vi "HFRR ADV v042.vi"() -> ()   [LabVIEW 2025] (continued)
                n3163 = local read "TITTLE"() -> (w3926:string)
                n3164 = call-dynamic "Set Report Header Text.vi"("report in"=w3909, "center header text"=w3926, "error in (no error)"=w3908) -> ("report out"=w3947:refnum<class "NI_report.lvclass">, "error out"=w3946:errorcluster)  [unwired: 11 in]
                n3165 = for {
                  N: 1 -> [_]
                  tunnel: [w3985] -> w3933
                  tunnel: [w3984] -> w3932
                  tunnel: w3947 -> [w3983]
                  tunnel: w3946 -> [w3982]
                  n3166 = call-dynamic "New Report Line.vi"("report in"=w3983, "error in (no error)"=w3982) -> ("report out"=w3985:refnum<class "NI_report.lvclass">, "error out"=w3984:errorcluster)  [unwired: 12 in]
                }
                n3167 = for {
                  N: 2 -> [_]
                  tunnel: [w3977] -> w3939
                  tunnel: [w3976] -> w3938
                  tunnel: w3933 -> [w3975]
                  tunnel: w3932 -> [w3974]
                  n3168 = call-dynamic "New Report Line.vi"("report in"=w3975, "error in (no error)"=w3974) -> ("report out"=w3977:refnum<class "NI_report.lvclass">, "error out"=w3976:errorcluster)  [unwired: 12 in]
                }
                n3169 = for {
                  N: 25 -> [_]
                  tunnel: w3939 -> [w3973]
                  tunnel: w3938 -> [w3971]
                  tunnel: [w3972] -> w3942
                  tunnel: [w3970] -> w3941
                  n3170 = call-dynamic "Set Report Tab Width.vi"("report in"=w3973, "error in (no error)"=w3971) -> ("report out"=w3972:refnum<class "NI_report.lvclass">, "error out"=w3970:errorcluster)  [unwired: 12 in]
                }
                n3171 = control-ref of="Tab Control 9"() -> (w3937:refnum<vi>)
                n3172 = call-dynamic "Append Control Image to Report.vi"("report in"=w3942, "alignment (default)"=HTML_Report_Image_Alignment."ABSMIDDLE", "ctrl reference"=w3937, "error in (no error)"=w3941) -> ("report out"=w3936:refnum<class "NI_report.lvclass">, "error out"=w3935:errorcluster)  [unwired: 8 in, 2 out]
                n3173 = for {
                  N: 3 -> [_]
                  tunnel: [w3969] -> w3920
                  tunnel: [w3968] -> w3919
                  tunnel: w3936 -> [w3967]
                  tunnel: w3935 -> [w3966]
                  n3174 = call-dynamic "New Report Line.vi"("report in"=w3967, "error in (no error)"=w3966) -> ("report out"=w3969:refnum<class "NI_report.lvclass">, "error out"=w3968:errorcluster)  [unwired: 12 in]
                }
                n3175 = for {
                  N: 100 -> [_]
                  tunnel: w3920 -> [w3965]
                  tunnel: w3919 -> [w3963]
                  tunnel: [w3964] -> w3916
                  tunnel: [w3962] -> w3914
                  n3176 = call-dynamic "Set Report Tab Width.vi"("report in"=w3965, "error in (no error)"=w3963) -> ("report out"=w3964:refnum<class "NI_report.lvclass">, "error out"=w3962:errorcluster)  [unwired: 12 in]
                }
                n3177 = String To Path(string="C:\\LAB-IQ\\im\\Temp_resized.jpg") -> (path=w3906:path)
                n3178 = call-poly <vilib>:"Append Image to Report.vi"("report in"=w3916, "path or URL of image"=w3906, "error in (no error)"=w3914) -> ("report out"=w3915:refnum<class "NI_report.lvclass">, "error out"=w3913:errorcluster)  [unwired: 9 in, 2 out]
                n3179 = call-poly <vilib>:"Open HTML Report in Browser.vi"("report in"=w3915, "error in (no error)"=w3913) -> ("report out"=w3950:refnum<class "NI_report.lvclass">, "error out"=w3949:errorcluster)  [unwired: 11 in, 1 out]
                n3180 = call-dynamic "Dispose Report.vi"("report in"=w3950, "error in (no error)"=w3949) -> ()  [unwired: 13 in, 1 out]
              }
              frame #2 {
              }
              frame #3 {
                n3181 = disable-structure shown="Disabled" {
                  frame Disabled {
                    n3182 = local read "String 10"() -> (w3990:string)
                    n3183 = Concatenate Strings("C:\\LAB-IQ-NXT\\Data\\" ("string"), w3990, ".jpg" ("string")) -> (w3988:string)
                    n3184 = String To Path(string=w3988) -> (path=w3987:path)
                    n3185 = Delete(path (use dialog)=w3987) -> ()  [unwired: 4 in, 3 out]
                  }
                  frame Enabled {
                  }
                }
                n3186 = local write "Print 2"(FALSE ("Print")) -> ()
              }
            }
          }
        }
      }
    }
    n3187 = Wait (ms)(milliseconds to wait=u32 50) -> ()  [unwired: 1 out]
    n3188 = Wait (ms)(milliseconds to wait=u32 50) -> ()  [unwired: 1 out]
    n3189 = local read "Quit"() -> (w2332:bool)
  }
  n3190 = VISA Close(VISA resource name=w43, error in (no error)=w42) -> ()  [unwired: 1 out]
  n3191 = while {
    stop <- w4141 stop-if-true
    n3192 = local read "Auto Start Test"() -> (w4139:bool)
    n3193 = local read "RUN"() -> (w4138:bool)
    n3194 = Wait (ms)(milliseconds to wait=u32 1000) -> ()  [unwired: 1 out]
    n3195 = Or(x=w4138, y=w4139) -> (x .or. y?=w4137:bool)
    n3196 = case shown="True" w4137 {
      frame False {
      }
      frame True {
        n3197 = local read "LVDT STROKE Actual"() -> (w4142:dbl)
        n3198 = In Range and Coerce(upper limit=1.2, x=w4142, lower limit=0.6) -> (In Range?=w4145:bool)  [unwired: 1 out]
        n3199 = call-poly <vilib>:"Random Number (Range).vi"("lower bound (0)"=0.998 ("upper bound (100)"), "upper bound (100)"=1.003) -> ("number"=w4143:dbl)  [unwired: 9 in]
        n3200 = case shown="True" w4145 {
          tunnel: [w4150 w4151] -> w4144
          tunnel: w4143 -> [_ w4151]
          tunnel: w4142 -> [w4150 _]
          frame False {
          }
          frame True {
          }
        }
        "LVDT STROKE DISPLAY" <- w4144
      }
    }
    n3201 = local read "Quit"() -> (w4141:bool)
  }
  n3202 = while {
    tunnel: [w4168] -> w51
    shift-right: [w4161] -> _
    shift-left: 0.0 -> [w4164]
    shift-right: [w4160] -> _
    shift-left: 0.0 -> [w4163]
    shift-right: [w4159] -> _
    shift-left: 100.0 ("vc_cmd") -> [w4162]
    stop <- w4168 stop-if-true
    # "PID LOGIC"
    n3203 = local read "run test Calibration"() -> (w4156:bool)
    n3204 = local read "RUN"() -> (w4166:bool)
    n3205 = local read "Auto Start Temp"() -> (w4157:bool)
    n3206 = local read "Auto Start Test"() -> (w4165:bool)
    n3207 = local read "START TEMP"() -> (w4155:bool)
    n3208 = And(x=w4157, y=w4165) -> (x .and. y?=w4158:bool)
    n3209 = Or(x=w4166, y=w4158) -> (x .or. y?=w4167:bool)
    n3210 = And(x=w4167, y=w4155) -> (x .and. y?=w4154:bool)
    n3211 = And(x=w4156, y=w4155) -> (x .and. y?=w4153:bool)
    n3212 = Or(x=w4153, y=w4154) -> (x .or. y?=w4152:bool)
    n3213 = Wait (ms)(milliseconds to wait="milliseconds to wait") -> ()  [unwired: 1 out]
    n3214 = case shown="True" w4152 {
      tunnel: [400.0 ("out_vc_cmd") w4187] -> w4159
      tunnel: [w4171 w4189] -> w4160
      tunnel: [w4171 w4188] -> w4161
      tunnel: w4164 -> [_ w4178]
      tunnel: w4163 -> [_ w4177]
      tunnel: w4162 -> [_ w4176]
      tunnel: w4156 -> [_ w4172]
      frame False {
        w4171 = 0.0 ("error_out")
      }
      frame True {
        n3215 = case shown="True" w4172 {
          tunnel: [w4196 1.0] -> w4174
          frame False {
            n3216 = local read "Set Strk"() -> (w4195:dbl)
            n3217 = Add(x=w4195, y="Add up Stroke") -> (x+y=w4196:dbl)
          }
          frame True {
          }
        }
        n3218 = local read "LVDT STROKE"() -> (w4173:dbl)
        n3219 = formula code="// Zero-Hardcode Explicit Positional-Form PID Engine\n// Inputs: target_stroke, measured_stroke, dt, prev_error, integral_accumulator_in, prev_vc_cmd\n//         kp, ki, kd, max_step_change, max_amplitude, min_amplitude, startup_cmd\n// Outputs: vc_cmd, error_out, out_error, integral_accumulator_out, out_vc_cmd\n\n// 1. Calculate Tracking Error\nfloat current_error = target_stroke - measured_stroke;\nerror_out = current_error;\n\n// 2. Compute Proportional Term\nfloat p_term = kp * current_error;\n\n// 3. Compute Derivative Term\nfloat d_term = 0.0;\nif (dt > 0.0) {\n    d_term = kd * ((current_error - prev_error) / dt);\n}\n\n// 4. Update and Accumulate Integral Term\nfloat current_integral = integral_accumulator_in + (current_error * dt);\nfloat i_term = ki * current_integral;\n\n// 5. Calculate Ideal Target Command (Anchored by startup baseline)\nfloat ideal_command = startup_cmd + p_term + i_term + d_term;\n\n// 6. Apply Loop Rate Limiting FIRST \n// (Forces the command to climb gradually from prev_vc_cmd instead of jumping straight to max)\nfloat raw_adjustment = ideal_command - prev_vc_cmd;\n\nif (raw_adjustment > max_step_change) {\n    raw_adjustment = max_step_change;\n} else if (raw_adjustment < -max_step_change) {\n    raw_adjustment = -max_step_change;\n}\n\nfloat next_vc_cmd = prev_vc_cmd + raw_adjustment;\n\n// 7. Anti-Windup Protection & Final Output Safety Safeguard Clamping\n// (Back-calculating based on what we are ACTUALLY outputting)\nif (next_vc_cmd > max_amplitude) {\n    float excess = next_vc_cmd - max_amplitude;\n    if (ki > 0.0) {\n        current_integral -= excess / ki;\n    }\n    next_vc_cmd = max_amplitude;\n} else if (next_vc_cmd < min_amplitude) {\n    float excess = next_vc_cmd - min_amplitude;\n    if (ki > 0.0) {\n        current_integral -= excess / ki;\n    }\n    next_vc_cmd = min_amplitude;\n}\n\n// 8. Map to Shift Registers for memory persistence\nvc_cmd = next_vc_cmd;\nout_error = current_error;                   \nintegral_accumulator_out = current_integral;  \nout_vc_cmd = next_vc_cmd;"("target_stroke"=w4174, "measured_stroke"=w4173, "dt"="dt", "integral_accumulator_in"=w4177, "prev_error"=w4178, "prev_vc_cmd"=w4176, "kp"="kp", "ki"="ki", "kd"="kd", "max_step_change"="max_step_change", "max_amplitude"="max_amplitude", "min_amplitude"="min_amplitude", "startup_cmd"="startup_cmd") -> ("vc_cmd"=w4193:dbl, "out_error"=w4188:dbl, "integral_accumulator_out"=w4189:dbl, "out_vc_cmd"=w4187:dbl)  [unwired: 1 out]
        "output Vpp" <- w4193
        n3220 = Number To Fractional String(number=w4193, precision (6)=i16 1) -> (F-format string=w4191:string)  [unwired: 2 in]
        n3221 = Concatenate Strings("DAC;" ("string"), w4191) -> (w4175:string)
        n3222 = local write "Due Write"(w4175) -> ()
        "prev_error" <- w4178
        "integral_accumulator_in" <- w4177
        "prev_vc_cmd" <- w4176
      }
    }
    n3223 = local read "Quit"() -> (w4168:bool)
  }
  n3224 = Or(x=w47, y=w46) -> (x .or. y?=w48:bool)
  n3225 = Or(x=w44, y=w48) -> (x .or. y?=w53:bool)
  n3226 = control-ref of="new picture"() -> ()  [unwired: 1 out]
  n3227 = Or(x=w56, y=w53) -> (x .or. y?=w50:bool)
  n3228 = Or(x=w50, y=w51) -> (x .or. y?=w45:bool)
  n3229 = while {
    tunnel: [w4198] -> w55
    i -> [w4205]
    stop <- w4198 stop-if-true
    n3230 = local read "Quit"() -> (w4198:bool)
    n3231 = Equal To 0?(x=w4205) -> (x = 0?=w4203:bool)
    n3232 = call "Elapsed Time3"("Time Target (s)"=45.0, "Auto Reset"=TRUE) -> ("Time has Elapsed"=w4202:bool)  [unwired: 10 in, 7 out]
    n3233 = Wait (ms)(milliseconds to wait=u32 50) -> ()  [unwired: 1 out]
    n3234 = Or(x=w4202, y=w4203) -> (x .or. y?=w4204:bool)
    n3235 = case shown="True" w4204 {
      frame False {
      }
      frame True {
        n3236 = call <vilib>:"System Exec.vi"("run minimized? (F)"=TRUE, "error in (no error)"="error in (no error)", "command line"="powercfg.exe -change -monitor-timeout-ac 0") -> ("error out"=w4216:errorcluster)  [unwired: 5 in, 3 out]
        n3237 = call <vilib>:"System Exec.vi"("run minimized? (F)"=TRUE, "error in (no error)"=w4216, "command line"="powercfg.exe -change -disk-timeout-ac 0") -> ("error out"=w4215:errorcluster)  [unwired: 5 in, 3 out]
        n3238 = call <vilib>:"System Exec.vi"("run minimized? (F)"=TRUE, "error in (no error)"=w4215, "command line"="powercfg.exe -change -standby-timeout-ac 0") -> ("error out"=w4214:errorcluster)  [unwired: 5 in, 3 out]
        n3239 = call <vilib>:"System Exec.vi"("run minimized? (F)"=TRUE, "error in (no error)"=w4214, "command line"="powercfg.exe -change -hibernate-timeout-ac 0") -> ("error out"=w4213:errorcluster)  [unwired: 5 in, 3 out]
        n3240 = call <vilib>:"Simple Error Handler.vi"("error in (no error)"=w4213) -> ("error out"=w4219:errorcluster)  [unwired: 4 in, 4 out]
        n3241 = call <vilib>:"Clear Errors.vi"("error in (no error)"=w4219) -> ("error out"=→"error out":errorcluster)  [unwired: 5 in, 1 out]
      }
    }
  }
  n3242 = Compound Arithmetic op=OR(w58, w45, w55) -> (w57:bool)
  n3243 = flat-sequence {
    tunnel: w57 -> [_]
    tunnel: [w4221] -> w27
    tunnel: w27 -> [_]
    frame #0 {
      n3244 = call "CLOSE CONNECTION.vi"() -> ("error out"=w4221:errorcluster)  [unwired: 11 in]
    }
    frame #1 {
      n3245 = Quit LabVIEW(quit? (T)=TRUE) -> ()
      n3246 = local write "Quit"(FALSE ("EXIT")) -> ()
    }
  }
  n3247 = property on="Heater Button" class="Bool (strict)"("Visible"=TRUE) -> ()  [unwired: 2 in, 2 out]
  n3248 = while {
    tunnel: [w4228] -> _
    i -> [w4228]
    stop <- w4224 stop-if-true
    # "Langauage selection"
    n3249 = Equal?(x="Lan flag", y=22.0) -> ()  [unwired: 1 out]
    n3250 = disable-structure shown="Disabled" {
      frame Disabled {
        n3251 = stacked-sequence {
          frame #0 {
            n3252 = case shown="\"Russian\"" "Language Selection" {
              tunnel: [0 1] -> w4230
              frame "English", Default {
              }
              frame "Russian" {
              }
            }
            n3253 = for {
              N: 130 -> [_]
              tunnel: "Table" -> [w4239]
              tunnel: w4230 -> [w4238]
              i -> [w4237]
              n3254 = Index Array(array=w4239, index (row)=w4237, index (col)=w4238) -> (element=w4236:string)
              n3255 = case shown="1" w4237 {
                tunnel: w4236 -> [w4240 w4241 _ w4242 w4243 w4244 w4245 w4246 w4247 w4248 w4249 w4250 w4251 w4252 w4253 w4254 w4255 w4256 w4257 w4258 w4259 w4260 w4261 w4262 w4263 w4264 w4265 w4266 w4267 _ _ w4268 w4269 w4270 w4271 w4272 w4273 w4282 w4289 w4296 w4303 w4307 w4310 w4313 w4315 w4317 w4318 w4319 w4320 w4321 w4322 w4323 w4324 w4325 w4326 w4327 w4328 w4329 w4330 w4331 w4332 w4333 w4334 w4335 w4336 w4337 w4338 w4339 w4340 w4341 w4342 w4343 w4344 w4345 w4346 w4347 w4348 w4349 w4350 w4351 w4352 w4353 w4354 w4355 w4356 w4357 w4358 w4359 w4360 w4361 w4362 w4363 w4364 w4365 w4366 w4367 w4368 w4369 w4370 w4371 w4372 w4373 w4374 w4375 w4376 _ w4377 w4378 w4379 w4380 w4381 w4382 w4383 w4384 w4385 w4386 w4387 w4388 w4389 _ w4390 w4391 w4392 w4393 w4394 w4395 _]
                frame 0 {
                  n3256 = local write "S"(w4240) -> ()
                }
                frame 1 {
                  n3257 = local write "S 2"(w4241) -> ()
                }
                frame 2 {
                }
                frame 3 {
                  n3258 = local write "S 4"(w4242) -> ()
                }
                frame 4 {
                  n3259 = property on="FILE" class="Str"("Caption.Text"=w4243) -> ()  [unwired: 2 in, 2 out]
                }
                frame 5 {
                  n3260 = property on="Fuel Discription :" class="Str"("Caption.Text"=w4244) -> ()  [unwired: 2 in, 2 out]
                }
                frame 6 {
                  n3261 = property on="Remarks :" class="Str"("Caption.Text"=w4245) -> ()  [unwired: 2 in, 2 out]
                }
                frame 7 {
                  n3262 = property on="Save & Continue" class="Bool (strict)"("Boolean Text.Text"=w4246) -> ()  [unwired: 2 in, 2 out]
                }
                frame 8 {
                }
                frame 9 {
                  n3263 = property on="Set Hz" class="DigNum (strict)"("Caption.Text"=w4248) -> ()  [unwired: 2 in, 2 out]
                }
                frame 10 {
                }
                frame 11 {
                  n3264 = property on="NORMAL LOAD" class="DigNum (strict)"("Caption.Text"=w4250) -> ()  [unwired: 2 in, 2 out]
                }
                frame 12 {
                }
                frame 13 {
                  n3265 = property on="Set Temp" class="DigNum (strict)"("Caption.Text"=w4252) -> ()  [unwired: 2 in, 2 out]
                }
                frame 14 {
                  n3266 = local write "S 15"(w4253) -> ()
                }
                frame 15 {
                  n3267 = property on="Set Rh" class="DigNum (strict)"("Caption.Text"=w4254) -> ()  [unwired: 2 in, 2 out]
                }
                frame 16 {
                }
                frame 17 {
                  n3268 = local write "S 18"(w4256) -> ()
                }
                frame 18 {
                  "String 17" <- w4257
                }
                frame 19 {
                  n3269 = property on="test time" class="DigNum (strict)"("Caption.Text"=w4258) -> ()  [unwired: 2 in, 2 out]
                }
                frame 20 {
                  "String 18" <- w4259
                  "String 22" <- w4259
                }
                frame 21 {
                  n3270 = property on="Elapsed time" class="DigNum (strict)"("Caption.Text"=w4260) -> ()  [unwired: 2 in, 2 out]
                }
                frame 22 {
                  n3271 = property on="Samplingtime 2" class="DigNum (strict)"("Caption.Text"=w4261) -> ()  [unwired: 2 in, 2 out]
                }
                frame 23 {
                  "String 21" <- w4262
                }
                frame 24 {
                  n3272 = property on="Countdown" class="DigNum (strict)"("Caption.Text"=w4263) -> ()  [unwired: 2 in, 2 out]
                }
                frame 25 {
                  n3273 = property on="Countdown 2" class="DigNum (strict)"("Caption.Text"=w4264) -> ()  [unwired: 2 in, 2 out]
                }
                frame 26 {
                  n3274 = property on="Engage" class="Bool (strict)"("Boolean Text.Text"=w4265) -> ()  [unwired: 2 in, 2 out]
                }
                frame 27 {
                  n3275 = property on="Boolean  4" class="Bool (strict)"("Boolean Text.Text"=w4266) -> ()  [unwired: 2 in, 2 out]
                }
                frame 28 {
                  n3276 = property on="Test \nStatus" class="Bool (strict)"("Boolean Text.Text"=w4267) -> ()  [unwired: 2 in, 2 out]
                }
                frame 29 {
                }
                frame 30 {
                }
                frame 31 {
                }
                frame 32 {
                  n3277 = property on="RSTCOF" class="Bool"("Boolean Text.Text"=w4269) -> ()  [unwired: 2 in, 2 out]
                  n3278 = property on="RST FF" class="Bool"("Boolean Text.Text"=w4269) -> ()  [unwired: 2 in, 2 out]
                  n3279 = property on="RST TEMP" class="Bool"("Boolean Text.Text"=w4269) -> ()  [unwired: 2 in, 2 out]
                  n3280 = property on="RSTV1 3" class="Bool"("Boolean Text.Text"=w4269) -> ()  [unwired: 2 in, 2 out]
                  n3281 = property on="rstv2" class="Bool"("Boolean Text.Text"=w4269) -> ()  [unwired: 2 in, 2 out]
                  n3282 = property on="RSTV1 2" class="Bool"("Boolean Text.Text"=w4269) -> ()  [unwired: 2 in, 2 out]
                  n3283 = property on="RST CP" class="Bool"("Boolean Text.Text"=w4269) -> ()  [unwired: 2 in, 2 out]
                }
                frame 33 {
                  "S 61" <- w4270
                }
                frame 34 {
                  "String 23" <- w4271
                }
                frame 35 {
                  n3284 = property on="Rh Before" class="DigNum (strict)"("Caption.Text"=w4272) -> ()  [unwired: 2 in, 2 out]
                }
                frame 36 {
                  n3285 = Match Pattern(string=w4273, regular expression=",") -> (before substring=→"bs":string, after substring=→"as":string)  [unwired: 1 in, 2 out]
                  n3286 = property on="Rh After" class="DigNum (strict)"("Caption.Text"=w4273) -> ()  [unwired: 2 in, 2 out]
                }
                frame 37 {
                  n3287 = Match Pattern(string=w4282, regular expression=",") -> (before substring=w4281:string, after substring=w4280:string)  [unwired: 1 in, 2 out]
                  "bs" <- w4281
                  "as" <- w4280
                  n3288 = Concatenate Strings(w4281, w4280) -> (w4277:string)
                  n3289 = property on="Humidity before test 2" class="DigNum (strict)"("Caption.Text"=w4277) -> ()  [unwired: 2 in, 2 out]
                  n3290 = Concatenate Strings(w4277, "=" ("string")) -> (w4278:string)
                  n3291 = local write "S 38"(w4278) -> ()
                }
                frame 38 {
                  n3292 = Match Pattern(string=w4289, regular expression=",") -> (before substring=w4288:string, after substring=w4287:string)  [unwired: 1 in, 2 out]
                  "bs" <- w4288
                  "as" <- w4287
                  n3293 = Concatenate Strings(w4288, w4287) -> (w4284:string)
                  n3294 = property on="Humidity after test 2" class="DigNum (strict)"("Caption.Text"=w4284) -> ()  [unwired: 2 in, 2 out]
                  n3295 = Concatenate Strings(w4284, "=" ("string")) -> (w4286:string)
                  n3296 = local write "S 39"(w4286) -> ()
                }
                frame 39 {
                  n3297 = Match Pattern(string=w4296, regular expression=",") -> (before substring=w4295:string, after substring=w4294:string)  [unwired: 1 in, 2 out]
                  "bs" <- w4295
                  "as" <- w4294
                  n3298 = Concatenate Strings(w4295, w4294) -> (w4291:string)
                  n3299 = property on="Temperature before test 2" class="DigNum (strict)"("Caption.Text"=w4291) -> ()  [unwired: 2 in, 2 out]
                  n3300 = Concatenate Strings(w4291, "=" ("string")) -> (→"String 34":string)
                }
                frame 40 {
                  n3301 = Match Pattern(string=w4303, regular expression=",") -> (before substring=w4302:string, after substring=w4301:string)  [unwired: 1 in, 2 out]
                  "bs" <- w4302
                  "as" <- w4301
                  n3302 = Concatenate Strings(w4302, w4301) -> (w4298:string)
                  n3303 = property on="Temperature after test 2" class="DigNum (strict)"("Caption.Text"=w4298) -> ()  [unwired: 2 in, 2 out]
                  n3304 = Concatenate Strings(w4298, "=" ("string")) -> (→"String 35":string)
                  n3305 = property on="Temperature after test" class="DigNum (strict)"("Caption.Text"=w4298) -> ()  [unwired: 2 in, 2 out]
                }
                frame 41 {
                  n3306 = property on="AVP 2" class="DigNum (strict)"("Caption.Text"=w4307) -> ()  [unwired: 2 in, 2 out]
                  n3307 = Concatenate Strings(w4307, "=" ("string")) -> (→"String 36":string)
                }
                frame 42 {
                  n3308 = property on="MWSD 2" class="DigNum (strict)"("Caption.Text"=w4310) -> ()  [unwired: 2 in, 2 out]
                  n3309 = Concatenate Strings(w4310, "=" ("string")) -> (→"String 37":string)
                }
                frame 43 {
                  n3310 = property on="HCF 2" class="DigNum (strict)"("Caption.Text"=w4313) -> ()  [unwired: 2 in, 2 out]
                  n3311 = Concatenate Strings(w4313, "=" ("string")) -> (→"String 38":string)
                }
                frame 44 {
                  n3312 = Concatenate Strings(w4315, "=" ("string")) -> (→"String 39":string)
                  n3313 = property on="WS1.4 2" class="DigNum (strict)"("Caption.Text"=w4315) -> ()  [unwired: 2 in, 2 out]
                }
                frame 45 {
                }
                frame 46 {
                  n3314 = local write "S 47"(w4318) -> ()
                }
                frame 47 {
                  n3315 = local write "S 48"(w4319) -> ()
                }
                frame 48 {
                  n3316 = local write "S 49"(w4320) -> ()
                }
                frame 49 {
                  n3317 = local write "S 50"(w4321) -> ()
                }
                frame 50 {
                  n3318 = local write "S 51"(w4322) -> ()
                }
                frame 51 {
                  n3319 = local write "S 52"(w4323) -> ()
                }
                frame 52 {
                  n3320 = local write "S 53"(w4324) -> ()
                }
                frame 53 {
                  n3321 = local write "S 54"(w4325) -> ()
                }
                frame 54 {
                  n3322 = local write "S 55"(w4326) -> ()
                }
                frame 55 {
                  n3323 = local write "S 56"(w4327) -> ()
                }
                frame 56 {
                  n3324 = local write "S 57"(w4328) -> ()
                }
                frame 57 {
                  n3325 = local write "S 58"(w4329) -> ()
                }
                frame 58 {
                  n3326 = local write "S 59"(w4330) -> ()
                }
                frame 59 {
                  n3327 = local write "S 60"(w4331) -> ()
                }
                frame 60 {
                  n3328 = local write "S 62"(w4332) -> ()
                }
                frame 61 {
                  n3329 = local write "S 63"(w4333) -> ()
                }
                frame 62 {
                  n3330 = local write "S 64"(w4334) -> ()
                }
                frame 63 {
                  n3331 = local write "S 65"(w4335) -> ()
                }
                frame 64 {
                  n3332 = local write "S 66"(w4336) -> ()
                }
                frame 65 {
                  n3333 = local write "S 67"(w4337) -> ()
                }
                frame 66 {
                  n3334 = local write "S 68"(w4338) -> ()
                }
                frame 67 {
                  n3335 = local write "S 69"(w4339) -> ()
                }
                frame 68 {
                  n3336 = local write "S 70"(w4340) -> ()
                }
                frame 69 {
                  n3337 = local write "S 71"(w4341) -> ()
                }
                frame 70 {
                  n3338 = local write "S 72"(w4342) -> ()
                }
                frame 71 {
                  n3339 = local write "S 73"(w4343) -> ()
                }
                frame 72 {
                  n3340 = local write "S 74"(w4344) -> ()
                }
                frame 73 {
                  n3341 = local write "S 75"(w4345) -> ()
                }
                frame 74 {
                  n3342 = local write "S 76"(w4346) -> ()
                }
                frame 75 {
                  n3343 = local write "S 77"(w4347) -> ()
                }
                frame 76 {
                  n3344 = local write "S 78"(w4348) -> ()
                }
                frame 77 {
                  n3345 = local write "S 79"(w4349) -> ()
                }
                frame 79 {
                  n3346 = property on="Sample Temperature ( °C )" class="XYGraph (strict)"("Y Scale.Name Label.Text"=w4350) -> ()  [unwired: 2 in, 2 out]
                }
                frame 80 {
                  n3347 = local write "S 81"(w4351) -> ()
                  n3348 = property on="Humidity ( %RH )" class="XYGraph (strict)"("Y Scale.Name Label.Text"=w4351) -> ()  [unwired: 2 in, 2 out]
                }
                frame 78 {
                  n3349 = property on="Air Temperature  ( °C )" class="XYGraph (strict)"("X Scale.Name Label.Text"=w4352) -> ()  [unwired: 2 in, 2 out]
                  n3350 = property on="Humidity ( %RH )" class="XYGraph (strict)"("X Scale.Name Label.Text"=w4352) -> ()  [unwired: 2 in, 2 out]
                  n3351 = property on="Sample Temperature ( °C )" class="XYGraph (strict)"("X Scale.Name Label.Text"=w4352) -> ()  [unwired: 2 in, 2 out]
                  n3352 = property on="Coefficient Of Friction" class="XYGraph (strict)"("X Scale.Name Label.Text"=w4352) -> ()  [unwired: 2 in, 2 out]
                }
                frame 81 {
                  n3353 = property on="Air Temperature  ( °C )" class="XYGraph (strict)"("Y Scale.Name Label.Text"=w4353) -> ()  [unwired: 2 in, 2 out]
                }
                frame 82 {
                  n3354 = local write "S 84"(w4354) -> ()
                }
                frame 83 {
                  n3355 = local write "S 85"(w4355) -> ()
                }
                frame 84 {
                  n3356 = local write "S 86"(w4356) -> ()
                }
                frame 85 {
                  n3357 = local write "S 87"(w4357) -> ()
                }
                frame 86 {
                  n3358 = local write "S 88"(w4358) -> ()
                }
                frame 87 {
                }
                frame 88 {
                  n3359 = local write "S 90"(w4360) -> ()
                }
                frame 89 {
                  n3360 = local write "S 91"(w4361) -> ()
                }
                frame 90 {
                  n3361 = local write "S 92"(w4362) -> ()
                }
                frame 91 {
                  n3362 = local write "S 93"(w4363) -> ()
                }
                frame 92 {
                  n3363 = local write "S 94"(w4364) -> ()
                }
                frame 93 {
                  n3364 = local write "S 95"(w4365) -> ()
                }
                frame 94 {
                  n3365 = local write "S 96"(w4366) -> ()
                }
                frame 95 {
                  n3366 = local write "S 97"(w4367) -> ()
                }
                frame 96 {
                  n3367 = local write "S 98"(w4368) -> ()
                }
                frame 97 {
                  n3368 = local write "S 99"(w4369) -> ()
                }
                frame 98 {
                  n3369 = local write "S 100"(w4370) -> ()
                }
                frame 99 {
                  n3370 = local write "S 101"(w4371) -> ()
                }
                frame 100 {
                  n3371 = local write "S 102"(w4372) -> ()
                }
                frame 101 {
                  n3372 = local write "S 103"(w4373) -> ()
                }
                frame 102 {
                  n3373 = local write "S 104"(w4374) -> ()
                }
                frame 103 {
                  n3374 = local write "S 105"(w4375) -> ()
                }
                frame 104 {
                  n3375 = local write "S 106"(w4376) -> ()
                }
                frame 105 {
                }
                frame 106 {
                  n3376 = property on="OK Button 17" class="Bool (strict)"("Boolean Text.Text"=w4377) -> ()  [unwired: 2 in, 2 out]
                }
                frame 107 {
                  n3377 = property on="OK Button 16" class="Bool (strict)"("Boolean Text.Text"=w4378) -> ()  [unwired: 2 in, 2 out]
                }
                frame 108 {
                  n3378 = property on="TITTLE" class="Str"("Caption.Text"=w4379) -> ()  [unwired: 2 in, 2 out]
                }
                frame 109 {
                  "String 30" <- w4380
                }
                frame 110 {
                  n3379 = property on="Test Date" class="Str"("Caption.Text"=w4381) -> ()  [unwired: 2 in, 2 out]
                  "String 31" <- w4381
                }
                frame 111 {
                  n3380 = property on="Sample ID" class="Str"("Caption.Text"=w4382) -> ()  [unwired: 2 in, 2 out]
                  "String 32" <- w4382
                }
                frame 112 {
                  n3381 = property on="Tested by" class="Str"("Caption.Text"=w4383) -> ()  [unwired: 2 in, 2 out]
                  "String 33" <- w4383
                }
                frame 113 {
                  n3382 = property on="System Configured Printers 2" class="Arr (strict)"("Caption.Text"=w4384) -> ()  [unwired: 2 in, 2 out]
                }
                frame 114 {
                  n3383 = property on="Selected Printer" class="Str"("Caption.Text"=w4385) -> ()  [unwired: 2 in, 2 out]
                }
                frame 115 {
                  n3384 = property on="Select Printer 3" class="DigNum (strict)"("Caption.Text"=w4386) -> ()  [unwired: 2 in, 2 out]
                }
                frame 116 {
                  n3385 = property on="Print" class="Bool (strict)"("Boolean Text.Text"=w4387) -> ()  [unwired: 2 in, 2 out]
                }
                frame 117 {
                  "String 41" <- w4388
                }
                frame 118 {
                  n3386 = property on="tested by" class="Str"("Caption.Text"=w4389) -> ()  [unwired: 2 in, 2 out]
                }
                frame 119 {
                }
                frame 120 {
                  n3387 = property on="Export" class="Bool (strict)"("Boolean Text.Text"=w4390) -> ()  [unwired: 2 in, 2 out]
                }
                frame 121 {
                }
                frame 122 {
                }
                frame 123 {
                  n3388 = property on="Select File Type" class="Enum (strict)"("Caption.Text"=w4393) -> ()  [unwired: 2 in, 2 out]
                }
                frame 124 {
                  n3389 = property on="s.NO" class="Str"("Caption.Text"=w4394) -> ()  [unwired: 2 in, 2 out]
                  "String 45" <- w4394
                }
                frame 125 {
                  n3390 = property on="trip1 8" class="Bool (strict)"("Boolean Text.Text"=w4395) -> ()  [unwired: 2 in, 2 out]
                }
                frame 126, Default {
                }
              }
            }
          }
          frame #1 {
            w4403 = TRUE ("Visible")
            n3391 = local read "S 91"() -> (w4420:string)
            n3392 = local read "S 90"() -> (w4419:string)
            n3393 = local read "S 88"() -> (w4418:string)
            n3394 = property on="File Path" class="Path"("Caption.Text"=w4419) -> ()  [unwired: 2 in, 2 out]
            n3395 = local read "S 71"() -> (w4413:string)
            n3396 = local read "S 86"() -> (w4415:string)
            n3397 = local read "S 85"() -> (w4416:string)
            n3398 = local read "S 87"() -> (w4414:string)
            n3399 = local read "S 84"() -> (w4417:string)
            n3400 = local read "S 103"() -> (w4402:string)
            n3401 = local read "S 104"() -> (w4401:string)
            n3402 = property on="Password" class="Str"("Caption.Text"=w4416) -> ()  [unwired: 2 in, 2 out]
            n3403 = property on="EDIT" class="Bool (strict)"("Boolean Text.Text"=w4413) -> ()  [unwired: 2 in, 2 out]
            n3404 = property on="SAVE" class="Bool (strict)"("Boolean Text.Text"=w4417) -> ()  [unwired: 2 in, 2 out]
            n3405 = Build Array(w4402, w4401) -> (w4400:string[])
            n3406 = property on="Heater Button" class="Bool (strict)"("Strings [4]"=w4400) -> ()  [unwired: 2 in, 2 out]
            n3407 = local read "S 92"() -> (w4412:string)
            n3408 = local read "S 93"() -> (w4411:string)
            n3409 = local read "S 105"() -> (w4398:string)
            n3410 = local read "S 106"() -> (w4397:string)
            n3411 = Build Array(w4412, w4411) -> ()  [unwired: 1 out]
            n3412 = Build Array(w4398, w4397) -> (w4399:string[])
            n3413 = local read "S 95"() -> (w4409:string)
            n3414 = local read "S 94"() -> (w4410:string)
            n3415 = local read "bs"() -> (w4425:string)
            n3416 = local read "as"() -> (w4426:string)
            n3417 = property on="Humidity" class="Bool (strict)"("Strings [4]"=w4399) -> ()  [unwired: 2 in, 2 out]
            n3418 = Concatenate Strings(w4425, "\r", w4426) -> ()  [unwired: 1 out]
            n3419 = property on="Rh After" class="DigNum (strict)"("Caption.Size to Text?"=TRUE ("Caption.Size to Text")) -> ()  [unwired: 2 in, 2 out]
            n3420 = local read "S 48"() -> (w4449:string)
            n3421 = local read "S 50"() -> (w4447:string)
            n3422 = local read "S 51"() -> (w4446:string)
            n3423 = local read "S 49"() -> (w4448:string)
            n3424 = local read "S 52"() -> (w4445:string)
            n3425 = local read "as"() -> (w4430:string)
            n3426 = local read "bs"() -> (w4431:string)
            n3427 = local read "S 56"() -> (w4444:string)
            n3428 = local read "S 57"() -> (w4443:string)
            n3429 = local read "S 58"() -> (w4442:string)
            n3430 = local read "S 59"() -> (w4441:string)
            n3431 = property on="OPEN" class="Bool (strict)"("Boolean Text.Text"=w4445) -> ()  [unwired: 2 in, 2 out]
            n3432 = property on="OPEN 1" class="Bool (strict)"("Boolean Text.Text"=w4449) -> ()  [unwired: 2 in, 2 out]
            n3433 = property on="OPEN 2" class="Bool (strict)"("Boolean Text.Text"=w4448) -> ()  [unwired: 2 in, 2 out]
            n3434 = property on="OPEN 3" class="Bool (strict)"("Boolean Text.Text"=w4447) -> ()  [unwired: 2 in, 2 out]
            n3435 = property on="OPEN 4" class="Bool (strict)"("Boolean Text.Text"=w4446) -> ()  [unwired: 2 in, 2 out]
            n3436 = Concatenate Strings(w4431, "\r", w4430) -> ()  [unwired: 1 out]
            n3437 = local read "S 102"() -> (w4404:string)
            n3438 = property on="КОФ1" class="DigNum (strict)"("Caption.Text"=w4444) -> ()  [unwired: 2 in, 2 out]
            n3439 = local read "S 98"() -> (w4408:string)
            n3440 = local read "S 99"() -> (w4407:string)
            n3441 = local read "S 100"() -> (w4406:string)
            n3442 = local read "S 101"() -> (w4405:string)
            n3443 = property on="КОФ2" class="DigNum (strict)"("Caption.Text"=w4443) -> ()  [unwired: 2 in, 2 out]
            n3444 = property on="КОФ3" class="DigNum (strict)"("Caption.Text"=w4442) -> ()  [unwired: 2 in, 2 out]
            n3445 = property on="КОФ4" class="DigNum (strict)"("Caption.Text"=w4441) -> ()  [unwired: 2 in, 2 out]
            n3446 = local read "bs"() -> (w4429:string)
            n3447 = local read "as"() -> (w4428:string)
            n3448 = local read "S 60"() -> (w4440:string)
            n3449 = local read "S 54"() -> (w4450:string)
            n3450 = Concatenate Strings(w4429, "\r", w4428) -> ()  [unwired: 1 out]
            n3451 = Concatenate Strings(w4450, w4440) -> ()  [unwired: 1 out]
            n3452 = local read "S 77"() -> (→"String 43":string)
            n3453 = local read "S 76"() -> (w4423:string)
            n3454 = local read "S 78"() -> (w4422:string)
            n3455 = local read "S 71"() -> (w4434:string)
            n3456 = local read "S 66"() -> (w4439:string)
            n3457 = local read "S 67"() -> (w4438:string)
            n3458 = local read "S 68"() -> (w4437:string)
            n3459 = local read "S 69"() -> (w4436:string)
            n3460 = local read "S 70"() -> (w4435:string)
            n3461 = property on="AIR TEMP" class="DigNum (strict)"("Caption.Text"=w4422) -> ()  [unwired: 2 in, 2 out]
            n3462 = property on="Set Strk" class="DigNum (strict)"("Caption.Text"=w4423) -> ()  [unwired: 2 in, 2 out]
            n3463 = property on="SPEED OUT:" class="DigNum (strict)"("Caption.Text"=w4437) -> ()  [unwired: 2 in, 2 out]
            n3464 = property on="EDIT" class="Bool (strict)"("Boolean Text.Text"=w4434) -> ()  [unwired: 2 in, 2 out]
            n3465 = local read "S 79"() -> (w4421:string)
          }
          frame #2 {
          }
        }
        n3466 = local write "Lan flag"(10.0 ("Lan flag")) -> ()
      }
      frame Enabled {
      }
    }
    n3467 = Wait (ms)(milliseconds to wait=u32 2000) -> ()  [unwired: 1 out]
    n3468 = local read "Quit"() -> (w4224:bool)
  }
  n3469 = while {
    shift-right: [w4456] -> _
    shift-left: _ -> [w4457]
    shift-right: [w4454] -> _
    shift-left: T18 {"Read Heave and Surge"="", "Bytes at Heave Port"=0.0, "Heave and Surge COM Port:"="COM9", "Com Port 2"="COM7", "Residual Due"="", "Heave COM Status 2"=TRUE, "Heave COM Status"=TRUE, "Port 2"=TRUE, "Sway PPR"=6400.0, "Surge PPR"=6400.0, "Heave PPR"=6400.0, "Sway Pitch"=2.0, "Surge Pitch"=3.0, "Heave Pitch"=4.0, "Sway Pulses/mm"=320.0, "Surge Pulses/mm"=1600.0, "Heave Pulses/mm"=1600.0, "inner loop"=0.0, "Read Heave and Surge 2"="", "String 36"="", "Write S"=FALSE, "WriteCC1"=[""], "Heave COM Loop"=0, "LastCom"="", "EXIT"=FALSE, "Error Heave"={"status"=TRUE, "code"=-1073807343, "source"=""}} -> [w4453]
    shift-right: [w4451] -> _
    shift-left: enum16{"init", "MAIN", "Panel Close"}."init" -> [w4452]
    stop <- w4455 stop-if-true
    # "HUMIDITY LOOP LOGIC"
    n3470 = case shown="\"MAIN\"" w4452 {
      tunnel: w4457 -> [w4471 w4495 w4559 w4561]
      tunnel: [w4466 w4482 w4559 w4561] -> w4456
      tunnel: [_ _ TRUE _] -> w4455
      tunnel: [w4463 w4480 w4557 w4560] -> w4454
      tunnel: w4453 -> [w4468 w4494 w4557 w4560]
      tunnel: [enum16{"init", "MAIN", "Panel Close"}."MAIN" w4489 _ _] -> w4451
      frame "init" {
        n3471 = local read "C3 :"() -> (w4458:refnum<visa-resource-name>)
        n3472 = Bundle By Name(cluster=w4468, "Heave and Surge COM Port:"=w4458) -> (w4467:T18)
        n3473 = call "Instrument fgv uno.vi"("Enum"=T31."INIT", "error in (no error) 2"=w4471, "INPUT"=w4467) -> ("error"=w4469:errorcluster, "output"=w4465:T18)  [unwired: 6 in, 1 out]
        n3474 = case shown="Error" w4469 {
          selector: w4469 -> [w4473 _]
          tunnel: [w4473 w4477] -> w4466
          tunnel: w4465 -> [w4472 w4475]
          tunnel: [w4472 w4474] -> w4464
          frame No Error {
          }
          frame Error {
            n3475 = call "Instrument fgv uno.vi"("Enum"=T31."ERROR INIT", "INPUT"=w4475) -> ("error"=w4478:errorcluster, "output"=w4474:T18)  [unwired: 7 in, 1 out]
            n3476 = call <vilib>:"Clear Errors.vi"("error in (no error)"=w4478) -> ("error out"=w4477:errorcluster)  [unwired: 5 in, 1 out]
          }
        }
        n3477 = local read "LastCom Humidity"() -> (w4461:string)
        n3478 = Unbundle By Name(w4464) -> ("Heave COM Status 2"=→"COM Status":bool, "Error Heave"=→"Error":errorcluster)  [unwired: 1 out]
        n3479 = Bundle By Name(cluster=w4464, "LastCom"=w4461) -> (w4463:T18)
      }
      frame "MAIN" {
        n3480 = Unbundle By Name(w4494) -> ("Com Port 2"=w4484:refnum<visa-resource-name>)
        n3481 = local read "C3 :"() -> (w4485:refnum<visa-resource-name>)
        n3482 = local write "COM Port Humidity :"(w4484) -> ()
        n3483 = Bundle By Name(cluster=w4494, "Heave and Surge COM Port:"=w4485) -> (w4493:T18)
        n3484 = Equal?(x=w4484, y=w4485) -> (x = y?=w4498:bool)
        n3485 = case shown="True" w4498 {
          tunnel: [w4513 w4530] -> w4483
          tunnel: w4495 -> [w4514 w4536]
          tunnel: w4493 -> [w4512 w4534]
          tunnel: [w4511 w4529] -> w4481
          frame False {
            n3486 = call <vilib>:"Clear Errors.vi"("error in (no error)"=w4514) -> ("error out"=w4510:errorcluster)  [unwired: 5 in, 1 out]
            n3487 = call "Instrument fgv uno.vi"("Enum"=T31."ERROR INIT", "error in (no error) 2"=w4510, "INPUT"=w4512) -> ("error"=w4516:errorcluster, "output"=w4511:T18)  [unwired: 6 in, 1 out]
            n3488 = call <vilib>:"Clear Errors.vi"("error in (no error)"=w4516) -> ("error out"=w4513:errorcluster)  [unwired: 5 in, 1 out]
          }
          frame True {
            n3489 = call "Instrument fgv uno.vi"("Enum"=T31."READ", "error in (no error) 2"=w4536, "INPUT"=w4534) -> ("error"=w4535:errorcluster, "output"=w4528:T18)  [unwired: 6 in, 1 out]
            n3490 = Bundle By Name(cluster=w4528, "String 36"="WRITE HUMIDITY") -> (w4527:T18)
            n3491 = case shown="True" "Write Humidity" {
              selector: "Write Humidity" -> [_ w4556]
              tunnel: w4535 -> [w4549 w4555]
              tunnel: [w4549 w4554] -> w4525
              tunnel: w4527 -> [w4548 w4552]
              tunnel: [w4548 w4551] -> w4524
              frame False {
              }
              frame True {
                n3492 = Not(x=w4556) -> (.not. x?=w4550:bool)
                n3493 = local write "Write Humidity"(w4550) -> ()
                n3494 = call "Instrument fgv uno.vi"("Enum"=T31."MANUAL WRITE", "error in (no error) 2"=w4555, "INPUT"=w4552) -> ("error"=w4554:errorcluster, "output"=w4551:T18)  [unwired: 6 in, 1 out]
              }
            }
            n3495 = Array Size(array="WriteHumidity") -> (size(s)=w4522:i32)
            n3496 = Greater Than 0?(x=w4522) -> (x > 0?=w4521:bool)
            n3497 = call "Instrument fgv uno.vi"("Enum"=T31."WRITE", "error in (no error) 2"=w4525, "WriteCC1"="WriteHumidity", "INPUT"=w4524) -> ("error"=w4532:errorcluster, "WriteCC1 2"=w4523:string[], "output"=w4531:T18)  [unwired: 5 in]
            n3498 = case shown="True" w4521 {
              tunnel: w4523 -> [_ w4538]
              frame False {
              }
              frame True {
                n3499 = local write "WriteHumidity"(w4538) -> ()
              }
            }
            n3500 = case shown="No Error" w4532 {
              selector: w4532 -> [w4539 w4542]
              tunnel: w4531 -> [w4540 w4547]
              tunnel: [w4540 w4546] -> w4529
              tunnel: [w4539 w4544] -> w4530
              frame No Error {
              }
              frame Error {
                n3501 = call <vilib>:"Clear Errors.vi"("error in (no error)"=w4542) -> ("error out"=w4541:errorcluster)  [unwired: 5 in, 1 out]
                n3502 = call "Instrument fgv uno.vi"("Enum"=T31."ERROR INIT", "error in (no error) 2"=w4541, "INPUT"=w4547) -> ("error"=w4545:errorcluster, "output"=w4546:T18)  [unwired: 6 in, 1 out]
                n3503 = call <vilib>:"Clear Errors.vi"("error in (no error)"=w4545) -> ("error out"=w4544:errorcluster)  [unwired: 5 in, 1 out]
              }
            }
            n3504 = Unbundle By Name(w4529) -> ("LastCom"=→"LastCom Humidity":string, "Read Heave and Surge"=→"Read HUMIDITY":string)
          }
        }
        n3505 = Unbundle By Name(w4481) -> ("Heave COM Status 2"=w4497:bool, "Error Heave"=w4486:errorcluster, "Bytes at Heave Port"=→"Bytes at Humidity Port  2":dbl)  [unwired: 1 out]
        n3506 = Unbundle By Name(w4486) -> ("status"=→"Humidity Port":bool)
        n3507 = Not(x=w4497) -> (.not. x?=w4487:bool)
        n3508 = local write "Error"(w4486) -> ()
        n3509 = local read "Quit"() -> (w4490:bool)
        n3510 = local write "COM Status"(w4487) -> ()
        n3511 = Select(t=enum16{"init", "MAIN", "Panel Close"}."Panel Close", s=w4490, f=enum16{"init", "MAIN", "Panel Close"}."MAIN") -> (s? t:f=w4489:enum16{"init", "MAIN", "Panel Close"})
        n3512 = local read "Humidity 2"() -> (w4479:bool)
        n3513 = case shown="True" w4479 {
          selector: w4479 -> [_ w4501]
          tunnel: w4483 -> [w4499 w4506]
          tunnel: [w4499 w4505] -> w4482
          tunnel: w4481 -> [w4500 w4504]
          tunnel: [w4500 w4503] -> w4480
          frame False {
          }
          frame True {
            n3514 = Not(x=w4501) -> (.not. x?=→"Humidity 2":bool)
            n3515 = call <vilib>:"Clear Errors.vi"("error in (no error)"=w4506) -> ("error out"=w4509:errorcluster)  [unwired: 5 in, 1 out]
            n3516 = call "Instrument fgv uno.vi"("Enum"=T31."ERROR INIT", "error in (no error) 2"=w4509, "INPUT"=w4504) -> ("error"=w4507:errorcluster, "output"=w4503:T18)  [unwired: 6 in, 1 out]
            n3517 = call <vilib>:"Clear Errors.vi"("error in (no error)"=w4507) -> ("error out"=w4505:errorcluster)  [unwired: 5 in, 1 out]
          }
        }
      }
      frame "Panel Close" {
      }
      frame Default {
      }
    }
  }
  n3518 = while {
    stop <- w4563 stop-if-true
    n3519 = call <vilib>:"High Resolution Polling Wait.vi"("seconds to wait"=0.05) -> ()  [unwired: 10 in, 1 out]
    n3520 = disable-structure shown="Enabled" {
      frame Disabled {
        n3521 = local read "Read HUMIDITY"() -> (w4564:string)
        n3522 = Spreadsheet String To Array(delimiter (Tab)=",", format string="", spreadsheet string=w4564, array type (2D Dbl)=string[] []) -> (array=w4583:string[])
        n3523 = for {
          tunnel: w4583 -> [w4592] mode=indexing
          tunnel: string[] ["STATE;", "SET;", "RH;", "T;", "AMB_RH;", "AMB_T;", "PUMP;", "FAN_IN;", "FAN_OUT;", "DEHUM;", "CURRENT;", "STALL;"] -> [w4591] mode=indexing
          tunnel: [w4590] -> w4582 mode=indexing
          n3524 = Match Pattern(string=w4592, regular expression=w4591) -> (after substring=w4590:string)  [unwired: 1 in, 3 out]
        }
        n3525 = Index Array(array=w4582) -> (element #1=w4581:string, element #2=w4580:string, element #3=w4572:string, element #4=w4571:string, element #5=w4570:string, element #6=w4579:string, element #7=w4578:string, element #8=w4577:string, element #9=w4576:string, element #10=w4575:string, element #11=w4574:string, element #12=w4573:string)  [unwired: 12 in]
        n3526 = Fract/Exp String To Number(string=w4572) -> (number=w4565:dbl)  [unwired: 3 in, 1 out]
        n3527 = Fract/Exp String To Number(string=w4570) -> (number=w4569:dbl)  [unwired: 3 in, 1 out]
        n3528 = local write "Ambient Humidity :"(w4569) -> ()
        n3529 = Equal?(x=w4565, y=0.0) -> (x = y?=w4567:bool)
        n3530 = case shown="True" w4567 {
          tunnel: [w4588 w4589] -> w4566
          tunnel: w4565 -> [w4588 _]
          frame False {
            (unwired) 0.0
            "Humidity temp" <- w4588
          }
          frame True {
            n3531 = local read "Humidity temp"() -> (w4589:dbl)
          }
        }
        "RH Numeric:" <- w4566
      }
      frame Enabled {
        n3532 = local read "Read HUMIDITY"() -> (w4612:string)
        n3533 = Spreadsheet String To Array(delimiter (Tab)=",", format string="", spreadsheet string=w4612, array type (2D Dbl)=dbl[] []) -> (array=w4608:dbl[])
        n3534 = Index Array(array=w4608) -> (element #1=→"STATE :":dbl, element #2=→"SET :":dbl, element #3=w4593:dbl, element #4=→"T :":dbl, element #5=→"AMB_RH :":dbl, element #6=→"AMB_T :":dbl, element #7=→"PUMP :":dbl, element #8=→"FAN_IN :":dbl, element #9=→"FAN_OUT :":dbl, element #10=→"DEHUM :":dbl, element #11=→"CURRENT :":dbl, element #12=→"STALL":dbl)  [unwired: 12 in]
        "RH :" <- w4593
        n3535 = Equal?(x=w4593, y=0.0) -> (x = y?=w4596:bool)
        n3536 = case shown="False" w4596 {
          tunnel: [w4613 w4614] -> w4597
          tunnel: w4593 -> [w4613 _]
          frame False {
            "Humidity temp 2" <- w4613
          }
          frame True {
            n3537 = local read "Humidity temp 2"() -> (w4614:dbl)
          }
        }
        n3538 = local write "RH Numeric:"(w4597) -> ()
      }
    }
    n3539 = local read "Quit"() -> (w4563:bool)
  }
  n3540 = while {
    shift-right: [w4620] -> _
    shift-left: _ -> [w4621]
    shift-right: [w4618] -> _
    shift-left: T20 {"Read Uno"="", "Bytes at Heave Port"=0.0, "UNO COM Port:"="COM9", "UNO COM Port: 2"="COM7", "Residual Due"="", "UNO COM Status 2"=TRUE, "UNO COM Status"=TRUE, "Port 2"=TRUE, "Sway PPR"=6400.0, "Surge PPR"=6400.0, "Heave PPR"=6400.0, "Sway Pitch"=2.0, "Surge Pitch"=3.0, "Heave Pitch"=4.0, "Sway Pulses/mm"=320.0, "Surge Pulses/mm"=1600.0, "Heave Pulses/mm"=1600.0, "inner loop"=0.0, "Read Heave and Surge 2"="", "String 36"="", "Write S"=FALSE, "WriteCC1"=[""], "Heave COM Loop"=0, "LastCom"="", "EXIT"=FALSE, "Error Heave"={"status"=TRUE, "code"=-1073807343, "source"=""}} -> [w4617]
    shift-right: [w4615] -> _
    shift-left: enum16{"init", "MAIN", "Panel Close"}."init" -> [w4616]
    stop <- w4619 stop-if-true
    # "UNO CODE LOGIC"
    n3541 = case shown="\"MAIN\"" w4616 {
      tunnel: w4621 -> [w4635 w4654 w4710 w4712]
      tunnel: [w4630 w4659 w4710 w4712] -> w4620
      tunnel: [_ _ TRUE _] -> w4619
      tunnel: [w4626 w4657 w4708 w4711] -> w4618
      tunnel: w4617 -> [w4632 w4653 w4708 w4711]
      tunnel: [enum16{"init", "MAIN", "Panel Close"}."MAIN" w4648 _ _] -> w4615
      frame "init" {
        n3542 = local read "Com Port 1"() -> (w4622:refnum<visa-resource-name>)
        n3543 = Bundle By Name(cluster=w4632, "UNO COM Port:"=w4622) -> (w4631:T20)
        n3544 = call "Instrument fgv.vi"("Enum"=T31."INIT", "error in (no error) 2"=w4635, "INPUT"=w4631) -> ("error"=w4633:errorcluster, "output"=w4629:T18)  [unwired: 6 in, 1 out]
        n3545 = case shown="Error" w4633 {
          selector: w4633 -> [w4637 _]
          tunnel: [w4637 w4641] -> w4630
          tunnel: w4629 -> [w4636 w4639]
          tunnel: [w4636 w4638] -> w4627
          frame No Error {
          }
          frame Error {
            n3546 = call "Instrument fgv.vi"("Enum"=T31."ERROR INIT", "INPUT"=w4639) -> ("error"=w4642:errorcluster, "output"=w4638:T18)  [unwired: 7 in, 1 out]
            n3547 = call <vilib>:"Clear Errors.vi"("error in (no error)"=w4642) -> ("error out"=w4641:errorcluster)  [unwired: 5 in, 1 out]
          }
        }
        n3548 = local read "LastCom UNO"() -> (w4624:string)
        n3549 = Unbundle By Name(w4627) -> ("Heave COM Status 2"=→"Instrument Status":bool, "Error Heave"=→"Error  2":errorcluster)  [unwired: 1 out]
        n3550 = Bundle By Name(cluster=w4627, "LastCom"=w4624) -> (w4626:T18)
      }
      frame "MAIN" {
        n3551 = Unbundle By Name(w4653) -> ("UNO COM Port: 2"=w4643:refnum<visa-resource-name>)
        n3552 = local read "Com Port 1"() -> (w4644:refnum<visa-resource-name>)
        n3553 = local write "COM Port UNO :"(w4643) -> ()
        n3554 = Equal?(x=w4643, y=w4644) -> (x = y?=w4660:bool)
        n3555 = Bundle By Name(cluster=w4653, "UNO COM Port:"=w4644) -> (w4652:T20)
        n3556 = case shown="True" w4660 {
          tunnel: [w4664 w4681] -> w4659
          tunnel: w4654 -> [w4665 w4687]
          tunnel: w4652 -> [w4663 w4685]
          tunnel: [w4662 w4680] -> w4657
          frame False {
            n3557 = call <vilib>:"Clear Errors.vi"("error in (no error)"=w4665) -> ("error out"=w4661:errorcluster)  [unwired: 5 in, 1 out]
            n3558 = call "Instrument fgv.vi"("Enum"=T31."ERROR INIT", "error in (no error) 2"=w4661, "INPUT"=w4663) -> ("error"=w4667:errorcluster, "output"=w4662:T18)  [unwired: 6 in, 1 out]
            n3559 = call <vilib>:"Clear Errors.vi"("error in (no error)"=w4667) -> ("error out"=w4664:errorcluster)  [unwired: 5 in, 1 out]
          }
          frame True {
            n3560 = call "Instrument fgv.vi"("Enum"=T31."READ", "error in (no error) 2"=w4687, "INPUT"=w4685) -> ("error"=w4686:errorcluster, "output"=w4679:T18)  [unwired: 6 in, 1 out]
            n3561 = Bundle By Name(cluster=w4679, "String 36"="WRITE UNO") -> (w4678:T18)
            n3562 = case shown="True" "Write" {
              selector: "Write" -> [_ w4702]
              tunnel: w4686 -> [w4700 w4707]
              tunnel: [w4700 w4706] -> w4676
              tunnel: w4678 -> [w4699 w4704]
              tunnel: [w4699 w4703] -> w4675
              frame False {
              }
              frame True {
                n3563 = Not(x=w4702) -> (.not. x?=w4701:bool)
                n3564 = local write "Write"(w4701) -> ()
                n3565 = call "Instrument fgv.vi"("Enum"=T31."MANUAL WRITE", "error in (no error) 2"=w4707, "INPUT"=w4704) -> ("error"=w4706:errorcluster, "output"=w4703:T18)  [unwired: 6 in, 1 out]
              }
            }
            n3566 = Array Size(array="Write UNO") -> (size(s)=w4673:i32)
            n3567 = Greater Than 0?(x=w4673) -> (x > 0?=w4672:bool)
            n3568 = call "Instrument fgv.vi"("Enum"=T31."WRITE", "error in (no error) 2"=w4676, "WriteCC1"="Write UNO", "INPUT"=w4675) -> ("error"=w4683:errorcluster, "WriteCC1 2"=w4674:string[], "output"=w4682:T18)  [unwired: 5 in]
            n3569 = case shown="True" w4672 {
              tunnel: w4674 -> [_ w4689]
              frame False {
              }
              frame True {
                n3570 = local write "Write UNO"(w4689) -> ()
              }
            }
            n3571 = case shown="Error" w4683 {
              selector: w4683 -> [w4690 w4693]
              tunnel: w4682 -> [w4691 w4698]
              tunnel: [w4691 w4697] -> w4680
              tunnel: [w4690 w4695] -> w4681
              frame No Error {
              }
              frame Error {
                n3572 = call <vilib>:"Clear Errors.vi"("error in (no error)"=w4693) -> ("error out"=w4692:errorcluster)  [unwired: 5 in, 1 out]
                n3573 = call "Instrument fgv.vi"("Enum"=T31."ERROR INIT", "error in (no error) 2"=w4692, "INPUT"=w4698) -> ("error"=w4696:errorcluster, "output"=w4697:T18)  [unwired: 6 in, 1 out]
                n3574 = call <vilib>:"Clear Errors.vi"("error in (no error)"=w4696) -> ("error out"=w4695:errorcluster)  [unwired: 5 in, 1 out]
              }
            }
            n3575 = Unbundle By Name(w4680) -> ("LastCom"=→"LastCom UNO":string, "Read Heave and Surge"=→"Read UNO":string)
          }
        }
        n3576 = Unbundle By Name(w4657) -> ("Heave COM Status 2"=w4658:bool, "Heave COM Status"=w4647:bool, "Error Heave"=w4645:errorcluster, "Bytes at Heave Port"=→"Bytes at Humidity Port":dbl)
        n3577 = Not(x=w4647) -> (.not. x?=w4655:bool)
        n3578 = Not(x=w4658) -> (.not. x?=w4646:bool)
        n3579 = local write "Instrument Status"(w4655) -> ()
        n3580 = local write "Error  2"(w4645) -> ()
        n3581 = local write "Port 1a"(w4647) -> ()
        n3582 = local read "Quit"() -> (w4649:bool)
        n3583 = local write "COM Status"(w4646) -> ()
        n3584 = Select(t=enum16{"init", "MAIN", "Panel Close"}."Panel Close", s=w4649, f=enum16{"init", "MAIN", "Panel Close"}."MAIN") -> (s? t:f=w4648:enum16{"init", "MAIN", "Panel Close"})
      }
      frame "Panel Close" {
      }
      frame Default {
      }
    }
  }
